vi "s.vi"() -> ()   [LabVIEW 2013] (continued)
      }
      event "OK Button 18": Value Change {
        n181 = event-data() -> ()  [unwired: 1 in, 6 out]
        n182 = Type Cast(x=0.0) -> (*(type *) &x=w670:string)  [unwired: 1 in]
        n183 = TCP Write(connection ID=w667, data in=w670, error in (no error)=w668) -> (connection ID out=w666:refnum<k5>, error out=w665:errorcluster)  [unwired: 1 in, 1 out]
        n184 = Bundle("OK Button 18"="OK Button 18", 16.0) -> (w674:cluster{"OK Button 18":bool, dbl})  [unwired: 1 in]
        n185 = Type Cast(x=w674) -> (*(type *) &x=w676:string)  [unwired: 1 in]
        n186 = TCP Write(connection ID=w666, data in=w676, error in (no error)=w665) -> (connection ID out=w673:refnum<k5>, error out=w672:errorcluster)  [unwired: 1 in, 1 out]
      }
      event Value Change {
        # "Air conditional - Bedroom 2"
        n187 = event-data() -> ()  [unwired: 1 in, 6 out]
        n188 = property on="Tab Control" class="TabCtl (strict)"("Visible"=FALSE) -> ()  [unwired: 2 in, 2 out]
        n189 = property on="Tab Control 2" class="TabCtl (strict)"("Visible"=FALSE) -> ()  [unwired: 2 in, 2 out]
        n190 = property on="Tab Control 3" class="TabCtl (strict)"("Visible"=FALSE) -> ()  [unwired: 2 in, 2 out]
        n191 = property on="Tab Control 4" class="TabCtl (strict)"("Visible"=FALSE) -> ()  [unwired: 2 in, 2 out]
        n192 = property on="Tab Control 5" class="TabCtl (strict)"("Visible"=FALSE) -> ()  [unwired: 2 in, 2 out]
        n193 = property on="Tab Control 11" class="TabCtl (strict)"("Visible"=FALSE) -> ()  [unwired: 2 in, 2 out]
        n194 = property on="Tab Control 6" class="TabCtl (strict)"("Visible"=FALSE) -> ()  [unwired: 2 in, 2 out]
        n195 = property on="Tab Control 10" class="TabCtl (strict)"("Visible"=FALSE) -> ()  [unwired: 2 in, 2 out]
        n196 = property on="Tab Control 13" class="TabCtl (strict)"("Visible"=FALSE) -> ()  [unwired: 2 in, 2 out]
        n197 = property on="Tab Control 7" class="TabCtl (strict)"("Visible"=FALSE) -> ()  [unwired: 2 in, 2 out]
        n198 = property on="Tab Control 12" class="TabCtl (strict)"("Visible"=FALSE) -> ()  [unwired: 2 in, 2 out]
        n199 = property on="Tab Control 8" class="TabCtl (strict)"("Visible"=FALSE) -> ()  [unwired: 2 in, 2 out]
        n200 = property on="Tab Control 9" class="TabCtl (strict)"("Visible"=FALSE) -> ()  [unwired: 2 in, 2 out]
        n201 = property on="Tab Control 24" class="TabCtl (strict)"("Visible"=FALSE) -> ()  [unwired: 2 in, 2 out]
        n202 = property on="Tab Control 15" class="TabCtl (strict)"("Visible"=FALSE) -> ()  [unwired: 2 in, 2 out]
        n203 = property on="Tab Control 21" class="TabCtl (strict)"("Visible"=TRUE) -> ()  [unwired: 2 in, 2 out]
        n204 = property on="Tab Control 16" class="TabCtl (strict)"("Visible"=FALSE) -> ()  [unwired: 2 in, 2 out]
        n205 = property on="Tab Control 17" class="TabCtl (strict)"("Visible"=FALSE) -> ()  [unwired: 2 in, 2 out]
        n206 = property on="Tab Control 22" class="TabCtl (strict)"("Visible"=FALSE) -> ()  [unwired: 2 in, 2 out]
        n207 = property on="Tab Control 23" class="TabCtl (strict)"("Visible"=FALSE) -> ()  [unwired: 2 in, 2 out]
        n208 = property on="Tab Control 18" class="TabCtl (strict)"("Visible"=FALSE) -> ()  [unwired: 2 in, 2 out]
        n209 = property on="Tab Control 19" class="TabCtl (strict)"("Visible"=FALSE) -> ()  [unwired: 2 in, 2 out]
        n210 = property on="Tab Control 14" class="TabCtl (strict)"("Visible"=FALSE) -> ()  [unwired: 2 in, 2 out]
      }
      event Value Change {
        n211 = event-data() -> ()  [unwired: 1 in, 6 out]
        n212 = Type Cast(x=0.0) -> (*(type *) &x=w705:string)  [unwired: 1 in]
        n213 = TCP Write(connection ID=w700, data in=w705, error in (no error)=w703) -> (connection ID out=w701:refnum<k5>, error out=w702:errorcluster)  [unwired: 1 in, 1 out]
        n214 = Bundle("?", 14.0) -> (w709:cluster{bool, dbl})  [unwired: 1 in]
        n215 = Type Cast(x=w709) -> (*(type *) &x=w711:string)  [unwired: 1 in]
        n216 = TCP Write(connection ID=w701, data in=w711, error in (no error)=w702) -> (connection ID out=w708:refnum<k5>, error out=w707:errorcluster)  [unwired: 1 in, 1 out]
      }
      event "OK Button 16": Value Change {
        n217 = event-data() -> ()  [unwired: 1 in, 6 out]
        n218 = Type Cast(x=0.0) -> (*(type *) &x=w717:string)  [unwired: 1 in]
        n219 = TCP Write(connection ID=w715, data in=w717, error in (no error)=w712) -> (connection ID out=w714:refnum<k5>, error out=w713:errorcluster)  [unwired: 1 in, 1 out]
        n220 = Bundle("OK Button 16"="OK Button 16", 20.0) -> (w721:cluster{"OK Button 16":bool, dbl})  [unwired: 1 in]
        n221 = Type Cast(x=w721) -> (*(type *) &x=w723:string)  [unwired: 1 in]
        n222 = TCP Write(connection ID=w714, data in=w723, error in (no error)=w713) -> (connection ID out=w720:refnum<k5>, error out=w719:errorcluster)  [unwired: 1 in, 1 out]
      }
      event Value Change {
        n223 = event-data() -> ()  [unwired: 1 in, 6 out]
        n224 = Type Cast(x=2.0) -> (*(type *) &x=w737:string)  [unwired: 1 in]
        n225 = TCP Write(connection ID=w728, data in=w737, error in (no error)=w727) -> (connection ID out=w735:refnum<k5>, error out=w734:errorcluster)  [unwired: 1 in, 1 out]
        n226 = Decimal String To Number(string="String") -> (number=w738:i32)  [unwired: 2 in, 1 out]
        n227 = Bundle(w738, 24.0, "?", 1.0) -> (w733:cluster{i32, dbl, bool, dbl})  [unwired: 1 in]
        n228 = Type Cast(x=w733) -> (*(type *) &x=w731:string)  [unwired: 1 in]
        n229 = TCP Write(connection ID=w735, data in=w731, error in (no error)=w734) -> (connection ID out=w729:refnum<k5>, error out=w730:errorcluster)  [unwired: 1 in, 1 out]
      }
      event Value Change {
        (unwired) FALSE ("Visible")
        n230 = event-data() -> ()  [unwired: 1 in, 6 out]
        n231 = property on="Tab Control 18" class="TabCtl (strict)"("Visible"=FALSE) -> ()  [unwired: 2 in, 2 out]
        n232 = property on="Tab Control 17" class="TabCtl (strict)"("Visible"=FALSE) -> ()  [unwired: 2 in, 2 out]
        n233 = property on="Tab Control 10" class="TabCtl (strict)"("Visible"=FALSE) -> ()  [unwired: 2 in, 2 out]
        n234 = property on="Tab Control 11" class="TabCtl (strict)"("Visible"=FALSE) -> ()  [unwired: 2 in, 2 out]
        n235 = property on="Tab Control 6" class="TabCtl (strict)"("Visible"=FALSE) -> ()  [unwired: 2 in, 2 out]
        n236 = property on="Tab Control 5" class="TabCtl (strict)"("Visible"=FALSE) -> ()  [unwired: 2 in, 2 out]
        n237 = property on="Tab Control 22" class="TabCtl (strict)"("Visible"=FALSE) -> ()  [unwired: 2 in, 2 out]
        n238 = property on="Tab Control 2" class="TabCtl (strict)"("Visible"=FALSE) -> ()  [unwired: 2 in, 2 out]
        n239 = property on="Tab Control 3" class="TabCtl (strict)"("Visible"=TRUE) -> ()  [unwired: 2 in, 2 out]
        n240 = property on="Tab Control 12" class="TabCtl (strict)"("Visible"=FALSE) -> ()  [unwired: 2 in, 2 out]
        n241 = property on="Tab Control 21" class="TabCtl (strict)"("Visible"=FALSE) -> ()  [unwired: 2 in, 2 out]
        n242 = property on="Tab Control 19" class="TabCtl (strict)"("Visible"=FALSE) -> ()  [unwired: 2 in, 2 out]
        n243 = property on="Tab Control 8" class="TabCtl (strict)"("Visible"=FALSE) -> ()  [unwired: 2 in, 2 out]
        n244 = property on="Tab Control 7" class="TabCtl (strict)"("Visible"=FALSE) -> ()  [unwired: 2 in, 2 out]
        n245 = property on="Tab Control 4" class="TabCtl (strict)"("Visible"=FALSE) -> ()  [unwired: 2 in, 2 out]
        n246 = property on="Tab Control 9" class="TabCtl (strict)"("Visible"=FALSE) -> ()  [unwired: 2 in, 2 out]
        n247 = property on="Tab Control" class="TabCtl (strict)"("Visible"=FALSE) -> ()  [unwired: 2 in, 2 out]
        n248 = property on="Tab Control 14" class="TabCtl (strict)"("Visible"=FALSE) -> ()  [unwired: 2 in, 2 out]
        n249 = property on="Tab Control 13" class="TabCtl (strict)"("Visible"=FALSE) -> ()  [unwired: 2 in, 2 out]
        n250 = property on="Tab Control 16" class="TabCtl (strict)"("Visible"=FALSE) -> ()  [unwired: 2 in, 2 out]
        n251 = property on="Tab Control 24" class="TabCtl (strict)"("Visible"=FALSE) -> ()  [unwired: 2 in, 2 out]
        n252 = property on="Tab Control 15" class="TabCtl (strict)"("Visible"=FALSE) -> ()  [unwired: 2 in, 2 out]
      }
      event Value Change {
        # "Air conditional - Bed room"
        n253 = event-data() -> ()  [unwired: 1 in, 6 out]
        n254 = local read item#4() -> (w761:dbl)
        n255 = Type Cast(x=5.0) -> (*(type *) &x=w767:string)  [unwired: 1 in]
        n256 = TCP Write(connection ID=w765, data in=w767, error in (no error)=w764) -> (connection ID out=w769:refnum<k5>, error out=w770:errorcluster)  [unwired: 1 in, 1 out]
        n257 = Bundle("?", w761, 3.0) -> (w771:cluster{bool, dbl, dbl})  [unwired: 1 in]
        n258 = Type Cast(x=w771) -> (*(type *) &x=w773:string)  [unwired: 1 in]
        n259 = TCP Write(connection ID=w769, data in=w773, error in (no error)=w770) -> (connection ID out=w763:refnum<k5>, error out=w762:errorcluster)  [unwired: 1 in, 1 out]
      }
      event Value Change {
        n260 = event-data() -> ()  [unwired: 1 in, 6 out]
        n261 = property on="Tab Control 18" class="TabCtl (strict)"("Visible"=FALSE) -> ()  [unwired: 2 in, 2 out]
        n262 = property on="Tab Control 17" class="TabCtl (strict)"("Visible"=FALSE) -> ()  [unwired: 2 in, 2 out]
        n263 = property on="Tab Control 10" class="TabCtl (strict)"("Visible"=FALSE) -> ()  [unwired: 2 in, 2 out]
        n264 = property on="Tab Control 6" class="TabCtl (strict)"("Visible"=FALSE) -> ()  [unwired: 2 in, 2 out]
        n265 = property on="Tab Control 5" class="TabCtl (strict)"("Visible"=FALSE) -> ()  [unwired: 2 in, 2 out]
        n266 = property on="Tab Control 2" class="TabCtl (strict)"("Visible"=FALSE) -> ()  [unwired: 2 in, 2 out]
        n267 = property on="Tab Control 3" class="TabCtl (strict)"("Visible"=FALSE) -> ()  [unwired: 2 in, 2 out]
        n268 = property on="Tab Control 22" class="TabCtl (strict)"("Visible"=FALSE) -> ()  [unwired: 2 in, 2 out]
        n269 = property on="Tab Control 12" class="TabCtl (strict)"("Visible"=FALSE) -> ()  [unwired: 2 in, 2 out]
        n270 = property on="Tab Control 8" class="TabCtl (strict)"("Visible"=FALSE) -> ()  [unwired: 2 in, 2 out]
        n271 = property on="Tab Control 7" class="TabCtl (strict)"("Visible"=FALSE) -> ()  [unwired: 2 in, 2 out]
        n272 = property on="Tab Control 4" class="TabCtl (strict)"("Visible"=FALSE) -> ()  [unwired: 2 in, 2 out]
        n273 = property on="Tab Control 21" class="TabCtl (strict)"("Visible"=FALSE) -> ()  [unwired: 2 in, 2 out]
        n274 = property on="Tab Control 9" class="TabCtl (strict)"("Visible"=FALSE) -> ()  [unwired: 2 in, 2 out]
        n275 = property on="Tab Control" class="TabCtl (strict)"("Visible"=FALSE) -> ()  [unwired: 2 in, 2 out]
        n276 = property on="Tab Control 11" class="TabCtl (strict)"("Visible"=FALSE) -> ()  [unwired: 2 in, 2 out]
        n277 = property on="Tab Control 19" class="TabCtl (strict)"("Visible"=FALSE) -> ()  [unwired: 2 in, 2 out]
        n278 = property on="Tab Control 24" class="TabCtl (strict)"("Visible"=FALSE) -> ()  [unwired: 2 in, 2 out]
        n279 = property on="Tab Control 16" class="TabCtl (strict)"("Visible"=TRUE) -> ()  [unwired: 2 in, 2 out]
        n280 = property on="Tab Control 14" class="TabCtl (strict)"("Visible"=FALSE) -> ()  [unwired: 2 in, 2 out]
        n281 = property on="Tab Control 13" class="TabCtl (strict)"("Visible"=FALSE) -> ()  [unwired: 2 in, 2 out]
        n282 = property on="Tab Control 15" class="TabCtl (strict)"("Visible"=FALSE) -> ()  [unwired: 2 in, 2 out]
      }
      event Value Change {
        n283 = event-data() -> ()  [unwired: 1 in, 6 out]
        n284 = property on="Tab Control 18" class="TabCtl (strict)"("Visible"=FALSE) -> ()  [unwired: 2 in, 2 out]
        n285 = property on="Tab Control 17" class="TabCtl (strict)"("Visible"=FALSE) -> ()  [unwired: 2 in, 2 out]
        n286 = property on="Tab Control 10" class="TabCtl (strict)"("Visible"=FALSE) -> ()  [unwired: 2 in, 2 out]
        n287 = property on="Tab Control 6" class="TabCtl (strict)"("Visible"=FALSE) -> ()  [unwired: 2 in, 2 out]
        n288 = property on="Tab Control 24" class="TabCtl (strict)"("Visible"=FALSE) -> ()  [unwired: 2 in, 2 out]
        n289 = property on="Tab Control 5" class="TabCtl (strict)"("Visible"=FALSE) -> ()  [unwired: 2 in, 2 out]
        n290 = property on="Tab Control 2" class="TabCtl (strict)"("Visible"=FALSE) -> ()  [unwired: 2 in, 2 out]
        n291 = property on="Tab Control 22" class="TabCtl (strict)"("Visible"=FALSE) -> ()  [unwired: 2 in, 2 out]
        n292 = property on="Tab Control 3" class="TabCtl (strict)"("Visible"=FALSE) -> ()  [unwired: 2 in, 2 out]
        n293 = property on="Tab Control 12" class="TabCtl (strict)"("Visible"=FALSE) -> ()  [unwired: 2 in, 2 out]
        n294 = property on="Tab Control 8" class="TabCtl (strict)"("Visible"=FALSE) -> ()  [unwired: 2 in, 2 out]
        n295 = property on="Tab Control 7" class="TabCtl (strict)"("Visible"=FALSE) -> ()  [unwired: 2 in, 2 out]
        n296 = property on="Tab Control 4" class="TabCtl (strict)"("Visible"=FALSE) -> ()  [unwired: 2 in, 2 out]
        n297 = property on="Tab Control 9" class="TabCtl (strict)"("Visible"=FALSE) -> ()  [unwired: 2 in, 2 out]
        n298 = property on="Tab Control 21" class="TabCtl (strict)"("Visible"=FALSE) -> ()  [unwired: 2 in, 2 out]
        n299 = property on="Tab Control" class="TabCtl (strict)"("Visible"=FALSE) -> ()  [unwired: 2 in, 2 out]
        n300 = property on="Tab Control 19" class="TabCtl (strict)"("Visible"=FALSE) -> ()  [unwired: 2 in, 2 out]
        n301 = property on="Tab Control 11" class="TabCtl (strict)"("Visible"=TRUE) -> ()  [unwired: 2 in, 2 out]
        n302 = property on="Tab Control 16" class="TabCtl (strict)"("Visible"=FALSE) -> ()  [unwired: 2 in, 2 out]
        n303 = property on="Tab Control 14" class="TabCtl (strict)"("Visible"=FALSE) -> ()  [unwired: 2 in, 2 out]
        n304 = property on="Tab Control 13" class="TabCtl (strict)"("Visible"=FALSE) -> ()  [unwired: 2 in, 2 out]
        n305 = property on="Tab Control 15" class="TabCtl (strict)"("Visible"=FALSE) -> ()  [unwired: 2 in, 2 out]
      }
      event Value Change {
        n306 = event-data() -> ()  [unwired: 1 in, 6 out]
        n307 = Type Cast(x=2.0) -> (*(type *) &x=w825:string)  [unwired: 1 in]
        n308 = TCP Write(connection ID=w821, data in=w825, error in (no error)=w820) -> (connection ID out=w827:refnum<k5>, error out=w828:errorcluster)  [unwired: 1 in, 1 out]
        n309 = Decimal String To Number(string="String") -> (number=w824:i32)  [unwired: 2 in, 1 out]
        n310 = Bundle(w824, 23.0, "?") -> (w829:cluster{i32, dbl, bool})  [unwired: 1 in]
        n311 = Type Cast(x=w829) -> (*(type *) &x=w831:string)  [unwired: 1 in]
        n312 = TCP Write(connection ID=w827, data in=w831, error in (no error)=w828) -> (connection ID out=w822:refnum<k5>, error out=w823:errorcluster)  [unwired: 1 in, 1 out]
      }
      event Value Change {
        n313 = event-data() -> ()  [unwired: 1 in, 6 out]
        n314 = property on="Tab Control 18" class="TabCtl (strict)"("Visible"=FALSE) -> ()  [unwired: 2 in, 2 out]
        n315 = property on="Tab Control 17" class="TabCtl (strict)"("Visible"=TRUE) -> ()  [unwired: 2 in, 2 out]
        n316 = property on="Tab Control 10" class="TabCtl (strict)"("Visible"=FALSE) -> ()  [unwired: 2 in, 2 out]
        n317 = property on="Tab Control 6" class="TabCtl (strict)"("Visible"=FALSE) -> ()  [unwired: 2 in, 2 out]
        n318 = property on="Tab Control 5" class="TabCtl (strict)"("Visible"=FALSE) -> ()  [unwired: 2 in, 2 out]
        n319 = property on="Tab Control 22" class="TabCtl (strict)"("Visible"=FALSE) -> ()  [unwired: 2 in, 2 out]
        n320 = property on="Tab Control 2" class="TabCtl (strict)"("Visible"=FALSE) -> ()  [unwired: 2 in, 2 out]
        n321 = property on="Tab Control 3" class="TabCtl (strict)"("Visible"=FALSE) -> ()  [unwired: 2 in, 2 out]
        n322 = property on="Tab Control 21" class="TabCtl (strict)"("Visible"=FALSE) -> ()  [unwired: 2 in, 2 out]
        n323 = property on="Tab Control 12" class="TabCtl (strict)"("Visible"=FALSE) -> ()  [unwired: 2 in, 2 out]
        n324 = property on="Tab Control 8" class="TabCtl (strict)"("Visible"=FALSE) -> ()  [unwired: 2 in, 2 out]
        n325 = property on="Tab Control 7" class="TabCtl (strict)"("Visible"=FALSE) -> ()  [unwired: 2 in, 2 out]
        n326 = property on="Tab Control 4" class="TabCtl (strict)"("Visible"=FALSE) -> ()  [unwired: 2 in, 2 out]
        n327 = property on="Tab Control 9" class="TabCtl (strict)"("Visible"=FALSE) -> ()  [unwired: 2 in, 2 out]
        n328 = property on="Tab Control" class="TabCtl (strict)"("Visible"=FALSE) -> ()  [unwired: 2 in, 2 out]
        n329 = property on="Tab Control 11" class="TabCtl (strict)"("Visible"=FALSE) -> ()  [unwired: 2 in, 2 out]
        n330 = property on="Tab Control 19" class="TabCtl (strict)"("Visible"=FALSE) -> ()  [unwired: 2 in, 2 out]
        n331 = property on="Tab Control 24" class="TabCtl (strict)"("Visible"=FALSE) -> ()  [unwired: 2 in, 2 out]
        n332 = property on="Tab Control 16" class="TabCtl (strict)"("Visible"=FALSE) -> ()  [unwired: 2 in, 2 out]
        n333 = property on="Tab Control 14" class="TabCtl (strict)"("Visible"=FALSE) -> ()  [unwired: 2 in, 2 out]
        n334 = property on="Tab Control 13" class="TabCtl (strict)"("Visible"=FALSE) -> ()  [unwired: 2 in, 2 out]
        n335 = property on="Tab Control 15" class="TabCtl (strict)"("Visible"=FALSE) -> ()  [unwired: 2 in, 2 out]
      }
      event Value Change {
        n336 = event-data() -> ()  [unwired: 1 in, 6 out]
        n337 = property on="Tab Control 18" class="TabCtl (strict)"("Visible"=TRUE) -> ()  [unwired: 2 in, 2 out]
        n338 = property on="Tab Control 17" class="TabCtl (strict)"("Visible"=FALSE) -> ()  [unwired: 2 in, 2 out]
        n339 = property on="Tab Control 24" class="TabCtl (strict)"("Visible"=FALSE) -> ()  [unwired: 2 in, 2 out]
        n340 = property on="Tab Control 10" class="TabCtl (strict)"("Visible"=FALSE) -> ()  [unwired: 2 in, 2 out]
        n341 = property on="Tab Control 6" class="TabCtl (strict)"("Visible"=FALSE) -> ()  [unwired: 2 in, 2 out]
        n342 = property on="Tab Control 5" class="TabCtl (strict)"("Visible"=FALSE) -> ()  [unwired: 2 in, 2 out]
        n343 = property on="Tab Control 22" class="TabCtl (strict)"("Visible"=FALSE) -> ()  [unwired: 2 in, 2 out]
        n344 = property on="Tab Control 2" class="TabCtl (strict)"("Visible"=FALSE) -> ()  [unwired: 2 in, 2 out]
        n345 = property on="Tab Control 3" class="TabCtl (strict)"("Visible"=FALSE) -> ()  [unwired: 2 in, 2 out]
        n346 = property on="Tab Control 12" class="TabCtl (strict)"("Visible"=FALSE) -> ()  [unwired: 2 in, 2 out]
        n347 = property on="Tab Control 8" class="TabCtl (strict)"("Visible"=FALSE) -> ()  [unwired: 2 in, 2 out]
        n348 = property on="Tab Control 7" class="TabCtl (strict)"("Visible"=FALSE) -> ()  [unwired: 2 in, 2 out]
        n349 = property on="Tab Control 4" class="TabCtl (strict)"("Visible"=FALSE) -> ()  [unwired: 2 in, 2 out]
        n350 = property on="Tab Control 9" class="TabCtl (strict)"("Visible"=FALSE) -> ()  [unwired: 2 in, 2 out]
        n351 = property on="Tab Control" class="TabCtl (strict)"("Visible"=FALSE) -> ()  [unwired: 2 in, 2 out]
        n352 = property on="Tab Control 21" class="TabCtl (strict)"("Visible"=FALSE) -> ()  [unwired: 2 in, 2 out]
        n353 = property on="Tab Control 11" class="TabCtl (strict)"("Visible"=FALSE) -> ()  [unwired: 2 in, 2 out]
        n354 = property on="Tab Control 19" class="TabCtl (strict)"("Visible"=FALSE) -> ()  [unwired: 2 in, 2 out]
        n355 = property on="Tab Control 16" class="TabCtl (strict)"("Visible"=FALSE) -> ()  [unwired: 2 in, 2 out]
        n356 = property on="Tab Control 14" class="TabCtl (strict)"("Visible"=FALSE) -> ()  [unwired: 2 in, 2 out]
        n357 = property on="Tab Control 13" class="TabCtl (strict)"("Visible"=FALSE) -> ()  [unwired: 2 in, 2 out]
        n358 = property on="Tab Control 15" class="TabCtl (strict)"("Visible"=FALSE) -> ()  [unwired: 2 in, 2 out]
      }
      event Value Change {
        n359 = event-data() -> ()  [unwired: 1 in, 6 out]
        n360 = Type Cast(x=1.0) -> (*(type *) &x=w876:string)  [unwired: 1 in]
        n361 = TCP Write(connection ID=w879, data in=w876, error in (no error)=w878) -> (connection ID out=w880:refnum<k5>, error out=w881:errorcluster)  [unwired: 1 in, 1 out]
        n362 = Bundle("?", 19.0) -> (w885:cluster{dbl, dbl})  [unwired: 1 in]
        n363 = Type Cast(x=w885) -> (*(type *) &x=w887:string)  [unwired: 1 in]
        n364 = TCP Write(connection ID=w880, data in=w887, error in (no error)=w881) -> (connection ID out=w883:refnum<k5>, error out=w882:errorcluster)  [unwired: 1 in, 1 out]
      }
      event Value Change {
        n365 = event-data() -> ()  [unwired: 1 in, 6 out]
        n366 = Type Cast(x=1.0) -> (*(type *) &x=w893:string)  [unwired: 1 in]
        n367 = TCP Write(connection ID=w890, data in=w893, error in (no error)=w889) -> (connection ID out=w895:refnum<k5>, error out=w896:errorcluster)  [unwired: 1 in, 1 out]
        n368 = Bundle("?", 21.0) -> (w897:cluster{dbl, dbl})  [unwired: 1 in]
        n369 = Type Cast(x=w897) -> (*(type *) &x=w899:string)  [unwired: 1 in]
        n370 = TCP Write(connection ID=w895, data in=w899, error in (no error)=w896) -> (connection ID out=w891:refnum<k5>, error out=w892:errorcluster)  [unwired: 1 in, 1 out]
      }
      event Value Change {
        n371 = event-data() -> ()  [unwired: 1 in, 6 out]
        n372 = Type Cast(x=1.0) -> (*(type *) &x=w905:string)  [unwired: 1 in]
        n373 = TCP Write(connection ID=w902, data in=w905, error in (no error)=w903) -> (connection ID out=w907:refnum<k5>, error out=w908:errorcluster)  [unwired: 1 in, 1 out]
        n374 = Bundle("?", 20.0) -> (w909:cluster{dbl, dbl})  [unwired: 1 in]
        n375 = Type Cast(x=w909) -> (*(type *) &x=w911:string)  [unwired: 1 in]
        n376 = TCP Write(connection ID=w907, data in=w911, error in (no error)=w908) -> (connection ID out=w901:refnum<k5>, error out=w900:errorcluster)  [unwired: 1 in, 1 out]
      }
      event Value Change {
        n377 = event-data() -> ()  [unwired: 1 in, 6 out]
        n378 = Type Cast(x=2.0) -> (*(type *) &x=w919:string)  [unwired: 1 in]
        n379 = TCP Write(connection ID=w916, data in=w919, error in (no error)=w915) -> (connection ID out=w921:refnum<k5>, error out=w922:errorcluster)  [unwired: 1 in, 1 out]
        n380 = Decimal String To Number(string="String") -> (number=w913:i32)  [unwired: 2 in, 1 out]
        n381 = Bundle(w913, 22.0, "?") -> (w923:cluster{i32, dbl, bool})  [unwired: 1 in]
        n382 = Type Cast(x=w923) -> (*(type *) &x=w925:string)  [unwired: 1 in]
        n383 = TCP Write(connection ID=w921, data in=w925, error in (no error)=w922) -> (connection ID out=w918:refnum<k5>, error out=w917:errorcluster)  [unwired: 1 in, 1 out]
      }
      event Value Change {
        (unwired) FALSE ("Visible")
        n384 = event-data() -> ()  [unwired: 1 in, 6 out]
        n385 = property on="Tab Control 18" class="TabCtl (strict)"("Visible"=FALSE) -> ()  [unwired: 2 in, 2 out]
        n386 = property on="Tab Control 17" class="TabCtl (strict)"("Visible"=FALSE) -> ()  [unwired: 2 in, 2 out]
        n387 = property on="Tab Control 6" class="TabCtl (strict)"("Visible"=FALSE) -> ()  [unwired: 2 in, 2 out]
        n388 = property on="Tab Control 10" class="TabCtl (strict)"("Visible"=FALSE) -> ()  [unwired: 2 in, 2 out]
        n389 = property on="Tab Control 8" class="TabCtl (strict)"("Visible"=FALSE) -> ()  [unwired: 2 in, 2 out]
        n390 = property on="Tab Control 9" class="TabCtl (strict)"("Visible"=FALSE) -> ()  [unwired: 2 in, 2 out]
        n391 = property on="Tab Control 19" class="TabCtl (strict)"("Visible"=FALSE) -> ()  [unwired: 2 in, 2 out]
        n392 = property on="Tab Control 5" class="TabCtl (strict)"("Visible"=FALSE) -> ()  [unwired: 2 in, 2 out]
        n393 = property on="Tab Control 22" class="TabCtl (strict)"("Visible"=FALSE) -> ()  [unwired: 2 in, 2 out]
        n394 = property on="Tab Control 7" class="TabCtl (strict)"("Visible"=FALSE) -> ()  [unwired: 2 in, 2 out]
        n395 = property on="Tab Control 12" class="TabCtl (strict)"("Visible"=FALSE) -> ()  [unwired: 2 in, 2 out]
        n396 = property on="Tab Control 21" class="TabCtl (strict)"("Visible"=FALSE) -> ()  [unwired: 2 in, 2 out]
        n397 = property on="Tab Control 11" class="TabCtl (strict)"("Visible"=FALSE) -> ()  [unwired: 2 in, 2 out]
        n398 = property on="Tab Control 4" class="TabCtl (strict)"("Visible"=TRUE) -> ()  [unwired: 2 in, 2 out]
        n399 = property on="Tab Control 3" class="TabCtl (strict)"("Visible"=FALSE) -> ()  [unwired: 2 in, 2 out]
        n400 = property on="Tab Control" class="TabCtl (strict)"("Visible"=FALSE) -> ()  [unwired: 2 in, 2 out]
        n401 = property on="Tab Control 2" class="TabCtl (strict)"("Visible"=FALSE) -> ()  [unwired: 2 in, 2 out]
        n402 = property on="Tab Control 14" class="TabCtl (strict)"("Visible"=FALSE) -> ()  [unwired: 2 in, 2 out]
        n403 = property on="Tab Control 13" class="TabCtl (strict)"("Visible"=FALSE) -> ()  [unwired: 2 in, 2 out]
        n404 = property on="Tab Control 24" class="TabCtl (strict)"("Visible"=FALSE) -> ()  [unwired: 2 in, 2 out]
        n405 = property on="Tab Control 15" class="TabCtl (strict)"("Visible"=FALSE) -> ()  [unwired: 2 in, 2 out]
        n406 = property on="Tab Control 16" class="TabCtl (strict)"("Visible"=FALSE) -> ()  [unwired: 2 in, 2 out]
      }
      event Value Change {
        n407 = event-data() -> ()  [unwired: 1 in, 6 out]
        n408 = property on="Tab Control 18" class="TabCtl (strict)"("Visible"=FALSE) -> ()  [unwired: 2 in, 2 out]
        n409 = property on="Tab Control 17" class="TabCtl (strict)"("Visible"=FALSE) -> ()  [unwired: 2 in, 2 out]
        n410 = property on="Tab Control 19" class="TabCtl (strict)"("Visible"=FALSE) -> ()  [unwired: 2 in, 2 out]
        n411 = property on="Tab Control 6" class="TabCtl (strict)"("Visible"=FALSE) -> ()  [unwired: 2 in, 2 out]
        n412 = property on="Tab Control 10" class="TabCtl (strict)"("Visible"=FALSE) -> ()  [unwired: 2 in, 2 out]
        n413 = property on="Tab Control 8" class="TabCtl (strict)"("Visible"=FALSE) -> ()  [unwired: 2 in, 2 out]
        n414 = property on="Tab Control 9" class="TabCtl (strict)"("Visible"=FALSE) -> ()  [unwired: 2 in, 2 out]
        n415 = property on="Tab Control 5" class="TabCtl (strict)"("Visible"=FALSE) -> ()  [unwired: 2 in, 2 out]
        n416 = property on="Tab Control 24" class="TabCtl (strict)"("Visible"=FALSE) -> ()  [unwired: 2 in, 2 out]
        n417 = property on="Tab Control 12" class="TabCtl (strict)"("Visible"=TRUE) -> ()  [unwired: 2 in, 2 out]
        n418 = property on="Tab Control 7" class="TabCtl (strict)"("Visible"=FALSE) -> ()  [unwired: 2 in, 2 out]
        n419 = property on="Tab Control 11" class="TabCtl (strict)"("Visible"=FALSE) -> ()  [unwired: 2 in, 2 out]
        n420 = property on="Tab Control 4" class="TabCtl (strict)"("Visible"=FALSE) -> ()  [unwired: 2 in, 2 out]
        n421 = property on="Tab Control 3" class="TabCtl (strict)"("Visible"=FALSE) -> ()  [unwired: 2 in, 2 out]
        n422 = property on="Tab Control" class="TabCtl (strict)"("Visible"=FALSE) -> ()  [unwired: 2 in, 2 out]
        n423 = property on="Tab Control 2" class="TabCtl (strict)"("Visible"=FALSE) -> ()  [unwired: 2 in, 2 out]
        n424 = property on="Tab Control 22" class="TabCtl (strict)"("Visible"=FALSE) -> ()  [unwired: 2 in, 2 out]
        n425 = property on="Tab Control 16" class="TabCtl (strict)"("Visible"=FALSE) -> ()  [unwired: 2 in, 2 out]
        n426 = property on="Tab Control 14" class="TabCtl (strict)"("Visible"=FALSE) -> ()  [unwired: 2 in, 2 out]
        n427 = property on="Tab Control 13" class="TabCtl (strict)"("Visible"=FALSE) -> ()  [unwired: 2 in, 2 out]
        n428 = property on="Tab Control 15" class="TabCtl (strict)"("Visible"=FALSE) -> ()  [unwired: 2 in, 2 out]
        n429 = property on="Tab Control 21" class="TabCtl (strict)"("Visible"=FALSE) -> ()  [unwired: 2 in, 2 out]
      }
      event Value Change {
        n430 = event-data() -> ()  [unwired: 1 in, 6 out]
        n431 = property on="Tab Control 14" class="TabCtl (strict)"("Visible"=FALSE) -> ()  [unwired: 2 in, 2 out]
        n432 = property on="Tab Control 13" class="TabCtl (strict)"("Visible"=TRUE) -> ()  [unwired: 2 in, 2 out]
        n433 = property on="Tab Control 19" class="TabCtl (strict)"("Visible"=FALSE) -> ()  [unwired: 2 in, 2 out]
        n434 = property on="Tab Control 6" class="TabCtl (strict)"("Visible"=FALSE) -> ()  [unwired: 2 in, 2 out]
        n435 = property on="Tab Control 15" class="TabCtl (strict)"("Visible"=FALSE) -> ()  [unwired: 2 in, 2 out]
        n436 = property on="Tab Control 10" class="TabCtl (strict)"("Visible"=FALSE) -> ()  [unwired: 2 in, 2 out]
        n437 = property on="Tab Control 8" class="TabCtl (strict)"("Visible"=FALSE) -> ()  [unwired: 2 in, 2 out]
        n438 = property on="Tab Control 9" class="TabCtl (strict)"("Visible"=FALSE) -> ()  [unwired: 2 in, 2 out]
        n439 = property on="Tab Control 5" class="TabCtl (strict)"("Visible"=FALSE) -> ()  [unwired: 2 in, 2 out]
        n440 = property on="Tab Control 22" class="TabCtl (strict)"("Visible"=FALSE) -> ()  [unwired: 2 in, 2 out]
        n441 = property on="Tab Control 12" class="TabCtl (strict)"("Visible"=FALSE) -> ()  [unwired: 2 in, 2 out]
        n442 = property on="Tab Control 7" class="TabCtl (strict)"("Visible"=FALSE) -> ()  [unwired: 2 in, 2 out]
        n443 = property on="Tab Control 11" class="TabCtl (strict)"("Visible"=FALSE) -> ()  [unwired: 2 in, 2 out]
        n444 = property on="Tab Control 4" class="TabCtl (strict)"("Visible"=FALSE) -> ()  [unwired: 2 in, 2 out]
        n445 = property on="Tab Control 3" class="TabCtl (strict)"("Visible"=FALSE) -> ()  [unwired: 2 in, 2 out]
        n446 = property on="Tab Control" class="TabCtl (strict)"("Visible"=FALSE) -> ()  [unwired: 2 in, 2 out]
        n447 = property on="Tab Control 2" class="TabCtl (strict)"("Visible"=FALSE) -> ()  [unwired: 2 in, 2 out]
        n448 = property on="Tab Control 24" class="TabCtl (strict)"("Visible"=FALSE) -> ()  [unwired: 2 in, 2 out]
        n449 = property on="Tab Control 16" class="TabCtl (strict)"("Visible"=FALSE) -> ()  [unwired: 2 in, 2 out]
        n450 = property on="Tab Control 21" class="TabCtl (strict)"("Visible"=FALSE) -> ()  [unwired: 2 in, 2 out]
        n451 = property on="Tab Control 18" class="TabCtl (strict)"("Visible"=FALSE) -> ()  [unwired: 2 in, 2 out]
        n452 = property on="Tab Control 17" class="TabCtl (strict)"("Visible"=FALSE) -> ()  [unwired: 2 in, 2 out]
      }
      event Value Change {
        n453 = event-data() -> ()  [unwired: 1 in, 6 out]
        n454 = property on="Tab Control 6" class="TabCtl (strict)"("Visible"=FALSE) -> ()  [unwired: 2 in, 2 out]
        n455 = property on="Tab Control 19" class="TabCtl (strict)"("Visible"=FALSE) -> ()  [unwired: 2 in, 2 out]
        n456 = property on="Tab Control 10" class="TabCtl (strict)"("Visible"=FALSE) -> ()  [unwired: 2 in, 2 out]
        n457 = property on="Tab Control 8" class="TabCtl (strict)"("Visible"=FALSE) -> ()  [unwired: 2 in, 2 out]
        n458 = property on="Tab Control 9" class="TabCtl (strict)"("Visible"=FALSE) -> ()  [unwired: 2 in, 2 out]
        n459 = property on="Tab Control 5" class="TabCtl (strict)"("Visible"=FALSE) -> ()  [unwired: 2 in, 2 out]
        n460 = property on="Tab Control 24" class="TabCtl (strict)"("Visible"=FALSE) -> ()  [unwired: 2 in, 2 out]
        n461 = property on="Tab Control 12" class="TabCtl (strict)"("Visible"=FALSE) -> ()  [unwired: 2 in, 2 out]
        n462 = property on="Tab Control 7" class="TabCtl (strict)"("Visible"=FALSE) -> ()  [unwired: 2 in, 2 out]
        n463 = property on="Tab Control 11" class="TabCtl (strict)"("Visible"=FALSE) -> ()  [unwired: 2 in, 2 out]
        n464 = property on="Tab Control 4" class="TabCtl (strict)"("Visible"=FALSE) -> ()  [unwired: 2 in, 2 out]
        n465 = property on="Tab Control 3" class="TabCtl (strict)"("Visible"=FALSE) -> ()  [unwired: 2 in, 2 out]
        n466 = property on="Tab Control" class="TabCtl (strict)"("Visible"=FALSE) -> ()  [unwired: 2 in, 2 out]
        n467 = property on="Tab Control 21" class="TabCtl (strict)"("Visible"=FALSE) -> ()  [unwired: 2 in, 2 out]
        n468 = property on="Tab Control 2" class="TabCtl (strict)"("Visible"=FALSE) -> ()  [unwired: 2 in, 2 out]
        n469 = property on="Tab Control 22" class="TabCtl (strict)"("Visible"=FALSE) -> ()  [unwired: 2 in, 2 out]
        n470 = property on="Tab Control 14" class="TabCtl (strict)"("Visible"=TRUE) -> ()  [unwired: 2 in, 2 out]
        n471 = property on="Tab Control 13" class="TabCtl (strict)"("Visible"=FALSE) -> ()  [unwired: 2 in, 2 out]
        n472 = property on="Tab Control 15" class="TabCtl (strict)"("Visible"=FALSE) -> ()  [unwired: 2 in, 2 out]
        n473 = property on="Tab Control 18" class="TabCtl (strict)"("Visible"=FALSE) -> ()  [unwired: 2 in, 2 out]
        n474 = property on="Tab Control 17" class="TabCtl (strict)"("Visible"=FALSE) -> ()  [unwired: 2 in, 2 out]
      }
      event Value Change {
        # "Air conditional - Master room"
        n475 = event-data() -> ()  [unwired: 1 in, 6 out]
        n476 = local read item#8() -> (w1013:dbl)
        n477 = Type Cast(x=5.0) -> (*(type *) &x=w1019:string)  [unwired: 1 in]
        n478 = TCP Write(connection ID=w1015, data in=w1019, error in (no error)=w1014) -> (connection ID out=w1021:refnum<k5>, error out=w1022:errorcluster)  [unwired: 1 in, 1 out]
        n479 = Bundle("?", w1013, 2.0) -> (w1023:cluster{bool, dbl, dbl})  [unwired: 1 in]
        n480 = Type Cast(x=w1023) -> (*(type *) &x=w1025:string)  [unwired: 1 in]
        n481 = TCP Write(connection ID=w1021, data in=w1025, error in (no error)=w1022) -> (connection ID out=w1017:refnum<k5>, error out=w1016:errorcluster)  [unwired: 1 in, 1 out]
      }
      event Value Change {
        # "Air conditional - Master room (slider)"
        n482 = event-data() -> ()  [unwired: 1 in, 6 out]
        n483 = local read item#5() -> (w1030:bool)
        n484 = Type Cast(x=5.0) -> (*(type *) &x=w1032:string)  [unwired: 1 in]
        n485 = TCP Write(connection ID=w1026, data in=w1032, error in (no error)=w1027) -> (connection ID out=w1034:refnum<k5>, error out=w1035:errorcluster)  [unwired: 1 in, 1 out]
        n486 = Bundle(w1030, "?", 2.0) -> (w1036:cluster{bool, dbl, dbl})  [unwired: 1 in]
        n487 = Type Cast(x=w1036) -> (*(type *) &x=w1038:string)  [unwired: 1 in]
        n488 = TCP Write(connection ID=w1034, data in=w1038, error in (no error)=w1035) -> (connection ID out=w1029:refnum<k5>, error out=w1028:errorcluster)  [unwired: 1 in, 1 out]
      }
      event Value Change {
        # "Air conditional - Bed room  (slider)_"
        n489 = event-data() -> ()  [unwired: 1 in, 6 out]
        n490 = local read item#1() -> (w1041:bool)
        n491 = Type Cast(x=5.0) -> (*(type *) &x=w1045:string)  [unwired: 1 in]
        n492 = TCP Write(connection ID=w1043, data in=w1045, error in (no error)=w1042) -> (connection ID out=w1047:refnum<k5>, error out=w1048:errorcluster)  [unwired: 1 in, 1 out]
        n493 = Bundle(w1041, "?", 3.0) -> (w1049:cluster{bool, dbl, dbl})  [unwired: 1 in]
        n494 = Type Cast(x=w1049) -> (*(type *) &x=w1051:string)  [unwired: 1 in]
        n495 = TCP Write(connection ID=w1047, data in=w1051, error in (no error)=w1048) -> (connection ID out=w1040:refnum<k5>, error out=w1039:errorcluster)  [unwired: 1 in, 1 out]
      }
      event Value Change {
        n496 = event-data() -> ()  [unwired: 1 in, 6 out]
        n497 = property on="Tab Control" class="TabCtl (strict)"("Visible"=FALSE) -> ()  [unwired: 2 in, 2 out]
        n498 = property on="Tab Control 2" class="TabCtl (strict)"("Visible"=FALSE) -> ()  [unwired: 2 in, 2 out]
        n499 = property on="Tab Control 3" class="TabCtl (strict)"("Visible"=FALSE) -> ()  [unwired: 2 in, 2 out]
        n500 = property on="Tab Control 4" class="TabCtl (strict)"("Visible"=FALSE) -> ()  [unwired: 2 in, 2 out]
        n501 = property on="Tab Control 5" class="TabCtl (strict)"("Visible"=FALSE) -> ()  [unwired: 2 in, 2 out]
        n502 = property on="Tab Control 11" class="TabCtl (strict)"("Visible"=FALSE) -> ()  [unwired: 2 in, 2 out]
        n503 = property on="Tab Control 6" class="TabCtl (strict)"("Visible"=FALSE) -> ()  [unwired: 2 in, 2 out]
        n504 = property on="Tab Control 10" class="TabCtl (strict)"("Visible"=FALSE) -> ()  [unwired: 2 in, 2 out]
        n505 = property on="Tab Control 13" class="TabCtl (strict)"("Visible"=FALSE) -> ()  [unwired: 2 in, 2 out]
        n506 = property on="Tab Control 7" class="TabCtl (strict)"("Visible"=FALSE) -> ()  [unwired: 2 in, 2 out]
        n507 = property on="Tab Control 12" class="TabCtl (strict)"("Visible"=FALSE) -> ()  [unwired: 2 in, 2 out]
        n508 = property on="Tab Control 8" class="TabCtl (strict)"("Visible"=FALSE) -> ()  [unwired: 2 in, 2 out]
        n509 = property on="Tab Control 9" class="TabCtl (strict)"("Visible"=FALSE) -> ()  [unwired: 2 in, 2 out]
        n510 = property on="Tab Control 15" class="TabCtl (strict)"("Visible"=FALSE) -> ()  [unwired: 2 in, 2 out]
        n511 = property on="Tab Control 24" class="TabCtl (strict)"("Visible"=TRUE) -> ()  [unwired: 2 in, 2 out]
        n512 = property on="Tab Control 21" class="TabCtl (strict)"("Visible"=FALSE) -> ()  [unwired: 2 in, 2 out]
        n513 = property on="Tab Control 16" class="TabCtl (strict)"("Visible"=FALSE) -> ()  [unwired: 2 in, 2 out]
        n514 = property on="Tab Control 17" class="TabCtl (strict)"("Visible"=FALSE) -> ()  [unwired: 2 in, 2 out]
        n515 = property on="Tab Control 22" class="TabCtl (strict)"("Visible"=FALSE) -> ()  [unwired: 2 in, 2 out]
        n516 = property on="Tab Control 23" class="TabCtl (strict)"("Visible"=FALSE) -> ()  [unwired: 2 in, 2 out]
        n517 = property on="Tab Control 18" class="TabCtl (strict)"("Visible"=FALSE) -> ()  [unwired: 2 in, 2 out]
        n518 = property on="Tab Control 19" class="TabCtl (strict)"("Visible"=FALSE) -> ()  [unwired: 2 in, 2 out]
        n519 = property on="Tab Control 14" class="TabCtl (strict)"("Visible"=FALSE) -> ()  [unwired: 2 in, 2 out]
      }
      event "play": Value Change {
        n520 = event-data() -> ()  [unwired: 1 in, 6 out]
        n521 = local read "flag 7"() -> (w1075:u16)
        n522 = local read "channel"() -> (w1076:dbl)
        n523 = Equal?(x=w1075, y=w1076) -> (x = y?=w1082:bool)
        n524 = case shown="False" w1082 {
          tunnel: w1081 -> [w1086 w1103]
          tunnel: w1080 -> [w1091 w1106]
          tunnel: w1079 -> [w1090 w1107]
          tunnel: [w1089 w1105] -> w1078
          tunnel: [w1088 w1104] -> w1077
          tunnel: w1075 -> [w1084 _]
          frame False {
            n525 = To Double Precision Float(number=w1084) -> (double precision float=w1083:dbl)
            n526 = local read "flag 7"() -> (→"channel":u16)
            n527 = local read "URL"() -> (w1101:string)
            n528 = property class="IWMPPlayer4"(reference=w1086, "URL"=w1101) -> (reference out=w1100:refnum<k7>)  [unwired: 1 in, 1 out]
            n529 = property class="IWMPPlayer4"(reference=w1100) -> ("controls"=w1099:refnum<k7>)  [unwired: 1 in, 2 out]
            n530 = invoke class="IWMPControls" method="play"(reference=w1099) -> (reference out=w1098:refnum<k7>)  [unwired: 2 in, 2 out]
            n531 = Type Cast(x=8.0) -> (*(type *) &x=w1092:string)  [unwired: 1 in]
            n532 = TCP Write(connection ID=w1091, data in=w1092, error in (no error)=w1090) -> (connection ID out=w1094:refnum<k5>, error out=w1095:errorcluster)  [unwired: 1 in, 1 out]
            n533 = Close Reference(reference=w1098) -> ()  [unwired: 1 in, 1 out]
            n534 = Bundle(w1083, 1.0) -> (w1096:cluster{dbl, dbl})  [unwired: 1 in]
            n535 = Type Cast(x=w1096) -> (*(type *) &x=w1097:string)  [unwired: 1 in]
            n536 = TCP Write(connection ID=w1094, data in=w1097, error in (no error)=w1095) -> (connection ID out=w1089:refnum<k5>, error out=w1088:errorcluster)  [unwired: 1 in, 1 out]
          }
          frame True {
            n537 = property class="IWMPPlayer4"(reference=w1103) -> ("controls"=w1114:refnum<k7>)  [unwired: 1 in, 2 out]
            n538 = invoke class="IWMPControls" method="play"(reference=w1114) -> (reference out=w1115:refnum<k7>)  [unwired: 2 in, 2 out]
            n539 = Type Cast(x=7.0) -> (*(type *) &x=w1108:string)  [unwired: 1 in]
            n540 = TCP Write(connection ID=w1106, data in=w1108, error in (no error)=w1107) -> (connection ID out=w1110:refnum<k5>, error out=w1111:errorcluster)  [unwired: 1 in, 1 out]
            n541 = Bundle(2.0) -> (w1112:cluster{dbl})  [unwired: 1 in]
            n542 = Type Cast(x=w1112) -> (*(type *) &x=w1113:string)  [unwired: 1 in]
            n543 = Close Reference(reference=w1115) -> ()  [unwired: 1 in, 1 out]
            n544 = TCP Write(connection ID=w1110, data in=w1113, error in (no error)=w1111) -> (connection ID out=w1105:refnum<k5>, error out=w1104:errorcluster)  [unwired: 1 in, 1 out]
          }
        }
      }
      event "flag 7": Value Change {
        n545 = event-data() -> ()  [unwired: 1 in, 6 out]
        n546 = case shown="2" "flag 7" {
          frame 0, Default {
            "URL" <- "C:\\Users\\kiat\\Downloads\\asd.mp4" ("URL")
          }
          frame 1 {
            n547 = local write "URL"("C:\\Users\\kiat\\Downloads\\videoplayback.mp4" ("URL")) -> ()
          }
          frame 2 {
            n548 = local write "URL"("C:\\Users\\kiat\\Downloads\\wiggle.mp4" ("URL")) -> ()
          }
        }
      }
      event "backward": Value Change {
        n549 = event-data() -> ()  [unwired: 1 in, 6 out]
        n550 = Automation Open(Automation Refnum=w1132) -> (Automation Refnum=w1133:refnum<k7>)  [unwired: 3 in, 1 out]
        n551 = property class="IWMPPlayer4"(reference=w1133) -> ("controls"=w1134:refnum<k7>)  [unwired: 1 in, 2 out]
        n552 = invoke class="IWMPControls" method="fastReverse"(reference=w1134) -> (reference out=w1131:refnum<k7>)  [unwired: 2 in, 2 out]
        n553 = Type Cast(x=7.0) -> (*(type *) &x=w1125:string)  [unwired: 1 in]
        n554 = TCP Write(connection ID=w1123, data in=w1125, error in (no error)=w1122) -> (connection ID out=w1127:refnum<k5>, error out=w1128:errorcluster)  [unwired: 1 in, 1 out]
        n555 = Close Reference(reference=w1131) -> ()  [unwired: 1 in, 1 out]
        n556 = Bundle(5.0) -> (w1129:cluster{dbl})  [unwired: 1 in]
        n557 = Type Cast(x=w1129) -> (*(type *) &x=w1130:string)  [unwired: 1 in]
        n558 = TCP Write(connection ID=w1127, data in=w1130, error in (no error)=w1128) -> (connection ID out=w1121:refnum<k5>, error out=w1120:errorcluster)  [unwired: 1 in, 1 out]
      }
      event "foward": Value Change {
        n559 = event-data() -> ()  [unwired: 1 in, 6 out]
        n560 = Type Cast(x=7.0) -> (*(type *) &x=w1140:string)  [unwired: 1 in]
        n561 = TCP Write(connection ID=w1138, data in=w1140, error in (no error)=w1137) -> (connection ID out=w1142:refnum<k5>, error out=w1143:errorcluster)  [unwired: 1 in, 1 out]
        n562 = Bundle(6.0) -> (w1144:cluster{dbl})  [unwired: 1 in]
        n563 = Type Cast(x=w1144) -> (*(type *) &x=w1145:string)  [unwired: 1 in]
        n564 = TCP Write(connection ID=w1142, data in=w1145, error in (no error)=w1143) -> (connection ID out=w1136:refnum<k5>, error out=w1135:errorcluster)  [unwired: 1 in, 1 out]
        n565 = Automation Open(Automation Refnum=w1147) -> (Automation Refnum=w1148:refnum<k7>)  [unwired: 3 in, 1 out]
        n566 = property class="IWMPPlayer4"(reference=w1148) -> ("controls"=w1149:refnum<k7>)  [unwired: 1 in, 2 out]
        n567 = invoke class="IWMPControls" method="fastForward"(reference=w1149) -> (reference out=w1146:refnum<k7>)  [unwired: 2 in, 2 out]
        n568 = Close Reference(reference=w1146) -> ()  [unwired: 1 in, 1 out]
      }
      event "pause": Value Change {
        n569 = event-data() -> ()  [unwired: 1 in, 6 out]
        n570 = Automation Open(Automation Refnum=w1162) -> (Automation Refnum=w1161:refnum<k7>)  [unwired: 3 in, 1 out]
        n571 = property class="IWMPPlayer4"(reference=w1161) -> ("controls"=w1164:refnum<k7>)  [unwired: 1 in, 2 out]
        n572 = invoke class="IWMPControls" method="pause"(reference=w1164) -> (reference out=w1163:refnum<k7>)  [unwired: 2 in, 2 out]
        n573 = Type Cast(x=7.0) -> (*(type *) &x=w1155:string)  [unwired: 1 in]
        n574 = TCP Write(connection ID=w1150, data in=w1155, error in (no error)=w1151) -> (connection ID out=w1157:refnum<k5>, error out=w1158:errorcluster)  [unwired: 1 in, 1 out]
        n575 = Close Reference(reference=w1163) -> ()  [unwired: 1 in, 1 out]
        n576 = Bundle(3.0) -> (w1159:cluster{dbl})  [unwired: 1 in]
        n577 = Type Cast(x=w1159) -> (*(type *) &x=w1160:string)  [unwired: 1 in]
        n578 = TCP Write(connection ID=w1157, data in=w1160, error in (no error)=w1158) -> (connection ID out=w1153:refnum<k5>, error out=w1152:errorcluster)  [unwired: 1 in, 1 out]
      }
      event "add": Value Change {
        n579 = event-data() -> ()  [unwired: 1 in, 6 out]
        n580 = Read from Text File(file (use dialog)=w1166) -> (refnum out=w1167:refnum<file>, text=w1165:string)  [unwired: 3 in, 2 out]
        n581 = while {
          tunnel: w1165 -> [w1171]
          border: w1165 -> [_]
          stop <- w1169 stop-if-true
          n582 = feedback #1() -> (w1177:string)
          n583 = xnode "Match Regular Expression"("input string"=w1177, "regular expression"="\n") -> ("before match"=w1174:string, "after match"=w1178:string)  [unwired: 4 in, 3 out]
          n584 = feedback-in #1(w1178) -> ()
          n585 = Empty String/Path?(string/path=w1178) -> (empty?=w1168:bool)
          n586 = xnode "Match Regular Expression"("input string"=w1174, "regular expression"="-") -> ("before match"=w1175:string)  [unwired: 4 in, 4 out]